vi "Dresden R2R Sputter 03.02.2018 IY24.vi"() -> ()   [LabVIEW 2009] (continued)
      }
    }
    n7249 = VISA Write(VISA resource name=w10738, write buffer=bytes[3], error in (no error)=w10737) -> (VISA resource name out=w10764, error out=w10763)  [unwired: 1 out]
    n7250 = stacked-sequence {
      tunnel: [w11051] -> w10740
      tunnel: w10764 -> [w11051]
      tunnel: [w11050] -> w10739
      tunnel: w10763 -> [w11050]
      frame #0 {
        n7251 = Wait Until Next ms Multiple(millisecond multiple=i32? 40) -> ()  [unwired: 1 out]
      }
    }
    n7252 = property class="Instr"(reference=w10740, error in=w10739) -> (reference out=w10766, error out=w10765, "Serial Settings:Number of Bytes at Serial Port"=w10767)
    n7253 = VISA Read(VISA resource name=w10766, byte count=w10767, error in (no error)=w10765) -> (VISA resource name out=w10736, read buffer=w10741, error out=w10735)  [unwired: 1 out]
    n7254 = Match Pattern(string=w10741, regular expression="Á") -> (after substring=w10731)  [unwired: 4 out]
    n7255 = String To Byte Array(string=w10731) -> (unsigned byte array=w10754)
    n7256 = String Length(string=w10731) -> (length=w10675)
    n7257 = Index Array(array=w10754, index=i32? 3) -> (element=w10746)
    n7258 = Index Array(array=w10754, index=i32? 2) -> (element=w10749)
    n7259 = Index Array(array=w10754, index=i32? 1) -> (element=w10758)
    n7260 = Index Array(array=w10754, index=data[5B]) -> (element=w10756)
    n7261 = Not Equal To 0?(x=w10675) -> (x != 0?=w10732)
    n7262 = To Unsigned Long Integer(number=w10746) -> (unsigned 32bit integer=w10748)
    n7263 = To Unsigned Long Integer(number=w10749) -> (unsigned 32bit integer=w10751)
    n7264 = To Unsigned Long Integer(number=w10758) -> (unsigned 32bit integer=w10757)
    n7265 = To Unsigned Long Integer(number=w10756) -> (unsigned 32bit integer=w10742)
    n7266 = case shown="True" w10732 {
      tunnel: [w11043 w11045] -> w10734
      tunnel: [w11042 w11044] -> w10733
      tunnel: w10736 -> [w11043 w11047]
      tunnel: w10735 -> [w11042 w11046]
      frame #0 {
      }
      frame #1 {
        n7267 = VISA Write(VISA resource name=w11047, write buffer=bytes[1], error in (no error)=w11046) -> (VISA resource name out=w11045, error out=w11044)  [unwired: 1 out]
      }
    }
    n7268 = Multiply(x=i32? 256, y=w10748) -> (x*y=w10745)
    n7269 = Multiply(x=i32? 256, y=w10751) -> (x*y=w10744)
    n7270 = Multiply(x=i32? 256, y=w10757) -> (x*y=w10743)
    n7271 = Compound Arithmetic op=ADD(w10745, w10744, w10743, w10742) -> (w10721)
    n7272 = case shown="1" w10675 {
      tunnel: w10721 -> [_ w11023]
      frame #0 {
      }
      frame #1 {
        "Frequency" <- w11023
      }
    }
  }
  n7273 = stacked-sequence {
    frame #0 {
      # "TM3"
      n7274 = stacked-sequence {
        tunnel: [_ "Thickness_Monitor3"] -> w11454
        frame #0 {
          n7275 = Wait (ms)(milliseconds to wait=u32 500) -> ()  [unwired: 1 out]
        }
        frame #1 {
        }
      }
      n7276 = call-poly "VISA Configure Serial Port"("VISA resource name"=w11454, "baud rate (9600)"=u32 57600) -> ("VISA resource name out"=w11456:refnum<visa-resource-name>, "error out"=w11455:errorcluster)  [unwired: 12 in]
      n7277 = VISA Clear(VISA resource name=w11456, error in (no error)=w11455) -> (VISA resource name out=w11453:refnum<visa-resource-name>, error out=w11452:errorcluster)
      n7278 = while {
        stop <- FALSE stop-if-true
        n7279 = local read "Tm3_fail"() -> (w11464:bool)
        n7280 = Wait Until Next ms Multiple(millisecond multiple=u32 1000) -> ()  [unwired: 1 out]
        n7281 = case shown="False" w11464 {
          frame #0 {
            # "Rate"
            n7282 = local read "Snsr3_thick"() -> (w11507:dbl)
            n7283 = feedback #159() -> (w11508:dbl)  [unwired: 1 in]
            n7284 = Subtract(x=w11507, y=w11508) -> (x-y=w11488:dbl)
            n7285 = local read "Material_density 3"() -> (w11489:dbl)
            n7286 = local read "Z_factor3"() -> (w11490:dbl)
            n7287 = feedback #160() -> (w11504:dbl)  [unwired: 1 in]
            n7288 = feedback #161() -> (w11492:dbl)  [unwired: 1 in]
            n7289 = feedback #162() -> (w11493:dbl)  [unwired: 1 in]
            n7290 = Equal?(x=w11492, y=w11490) -> (x = y?=w11494:bool)
            n7291 = Equal?(x=w11493, y=w11489) -> (x = y?=w11495:bool)
            n7292 = feedback #163() -> (w11503:dbl)  [unwired: 1 in]
            n7293 = And(x=w11494, y=w11495) -> (x .and. y?=w11491:bool)
            n7294 = case shown="True" w11491 {
              tunnel: w11488 -> [_ w11523]
              tunnel: [0.0 w11523] -> w11487
              frame #0 {
                n7295 = Wait (ms)(milliseconds to wait=u32 2000) -> ()  [unwired: 1 out]
              }
              frame #1 {
              }
            }
            n7296 = feedback #164() -> (w11502:dbl)  [unwired: 1 in]
            n7297 = feedback #165() -> (w11501:dbl)  [unwired: 1 in]
            n7298 = feedback #166() -> (w11500:dbl)  [unwired: 1 in]
            n7299 = feedback #167() -> (w11499:dbl)  [unwired: 1 in]
            n7300 = feedback #168() -> (w11498:dbl)  [unwired: 1 in]
            n7301 = feedback #169() -> (w11497:dbl)  [unwired: 1 in]
            n7302 = feedback #170() -> (w11496:dbl)  [unwired: 1 in]
            n7303 = Compound Arithmetic op=ADD(w11487, w11504, w11503, w11502, w11501, w11500, w11499, w11498, w11497, w11496) -> (w11505:dbl)
            n7304 = Divide(x=w11505, y=10.0) -> (x/y=w11484:dbl)
            n7305 = Greater Or Equal?(x=w11484, y=0.0) -> (x >= y?=w11486:bool)
            n7306 = case shown="True" w11486 {
              tunnel: w11484 -> [w11513 _]
              frame #0 {
                # "kA"
                n7307 = Divide(x="Tooling_factor3", y=100.0) -> (x/y=w11514:dbl)
                n7308 = Multiply(x=w11514, y=w11513) -> (x*y=w11509:dbl)
                "Rate3-2" <- w11509
                "Rate3-1" <- w11509
                "Rate3-3" <- w11509
                "Rate3-4" <- w11509
                "Rate3-5" <- w11509
                n7309 = Divide(x=w11509, y=1000.0) -> (x/y=w11518:dbl)
                n7310 = local read "Thickness 3-1"() -> (w11519:dbl)
                n7311 = Add(x=w11519, y=w11518) -> (x+y=w11511:dbl)
                n7312 = Greater?(x=w11511, y=0.0) -> (0:w11516:bool)
                n7313 = case shown="True" w11516 {
                  tunnel: w11511 -> [_ w11520]
                  frame #0 {
                  }
                  frame #1 {
                    "Thickness 3-1" <- w11520
                    "Thickness 3-2" <- w11520
                    "Thickness 3-3" <- w11520
                  }
                }
              }
              frame #1 {
              }
            }
          }
          frame #1 {
            w11524 = 0.0 ("Rate1-1")
            n7314 = local write "Rate3-1"(w11524) -> ()
            n7315 = local write "Rate3-2"(w11524) -> ()
            n7316 = local write "Rate3-3"(w11524) -> ()
            n7317 = local write "Rate3-4"(w11524) -> ()
            n7318 = local write "Rate3-5"(w11524) -> ()
          }
        }
        n7319 = Compound Arithmetic op=OR("Tm3_auto_set_zero", "Set3_zero_parameter", "Set3_zero_parameter2") -> (w11460:bool)
        n7320 = case shown="True" w11460 {
          frame #0 {
          }
          frame #1 {
            w11479 = 0.0 ("Thickness 1-1")
            n7321 = local read "Start_coating"() -> (w11474:bool)
            n7322 = local read "Semi"() -> (w11475:bool)
            n7323 = local read "Loading"() -> (w11473:bool)
            n7324 = Compound Arithmetic op=OR(w11475, w11474, w11473) -> (w11476:bool)
            n7325 = case shown="False" w11476 {
              frame #0 {
                n7326 = stacked-sequence {
                  frame #0 {
                    n7327 = local write "Pps_code_entry"("" ("Pps_code_entry")) -> ()
                  }
                  frame #1 {
                    n7328 = Wait (ms)(milliseconds to wait=u32 500) -> ()  [unwired: 1 out]
                  }
                  frame #2 {
                    n7329 = local write "Ppsok"(TRUE ("Ppsok")) -> ()
                  }
                }
              }
              frame #1 {
              }
            }
            n7330 = local write "Set3_zero_parameter2"(FALSE ("Set1_zero_parameter 2")) -> ()
            n7331 = local write "Set3_zero_parameter"(FALSE ("Set1_zero_parameter")) -> ()
            n7332 = local write "Tm3_auto_set_zero"(FALSE ("Tm1_auto_set_zero")) -> ()
            n7333 = local write "Thickness 3-2"(w11479) -> ()
            n7334 = local write "Thickness 3-3"(w11479) -> ()
          }
        }
        n7335 = local read "Frequency_short3"() -> (w11459:u32)
        n7336 = Not Equal To 0?(x=w11459) -> (x != 0?=w11458:bool)
        n7337 = case shown="True" w11458 {
          frame #0 {
            n7338 = local write "Tm3_gui"(FALSE ("Tm1_fail")) -> ()
          }
          frame #1 {
            n7339 = local read "Thickness 3-1"() -> (w11470:dbl)
            n7340 = Greater?(x=w11470, y="Thickness_for_TM3_gui") -> (0:w11468:bool)
            n7341 = case shown="False" w11468 {
              frame #0 {
                n7342 = local write "Tm3_gui"(FALSE ("Tm1_fail")) -> ()
              }
              frame #1 {
                n7343 = local write "Tm3_gui"(TRUE ("Tm1_fail")) -> ()
              }
            }
          }
        }
      }
      n7344 = while {
        tunnel: w11453 -> [w11677]
        tunnel: w11452 -> [w11676]
        tunnel: [w11670] -> w11451
        tunnel: [w11669] -> w11450
        stop <- FALSE stop-if-true
        n7345 = Wait Until Next ms Multiple(millisecond multiple=u32 250) -> ()  [unwired: 1 out]
        n7346 = case shown="True" "Tm3_set_parameters" {
          frame #0 {
          }
          frame #1 {
            n7347 = stacked-sequence {
              frame #0 {
                n7348 = local write "Pps_code_entry"("" ("Pps_code_entry")) -> ()
              }
              frame #1 {
                n7349 = Wait (ms)(milliseconds to wait=u32 500) -> ()  [unwired: 1 out]
              }
              frame #2 {
                n7350 = local write "Ppsok"(TRUE ("Ppsok")) -> ()
              }
            }
          }
        }
        n7351 = VISA Write(VISA resource name=w11677, write buffer="ª\u0004È¡È\u0001S\u0001\u0000\u0000\u0000Š", error in (no error)=w11676) -> (VISA resource name out=w11679:refnum<visa-resource-name>, error out=w11680:errorcluster)  [unwired: 1 out]
        n7352 = property class="Instr"(reference=w11679, error in=w11680) -> (reference out=w11681:refnum<visa-resource-name>, error out=w11683:errorcluster, "Serial Settings:Number of Bytes at Serial Port"=w11682:u32)
        n7353 = stacked-sequence {
          tunnel: [w11810] -> w11684
          tunnel: w11681 -> [w11810]
          tunnel: [w11809] -> w11686
          tunnel: w11683 -> [w11809]
          tunnel: [w11808] -> w11685
          tunnel: w11682 -> [w11808]
          frame #0 {
            n7354 = Wait (ms)(milliseconds to wait=u32 100) -> ()  [unwired: 1 out]
          }
        }
        n7355 = VISA Read(VISA resource name=w11684, byte count=w11685, error in (no error)=w11686) -> (VISA resource name out=w11670:refnum<visa-resource-name>, read buffer=w11671:string, error out=w11669:errorcluster)  [unwired: 1 out]
        "Tm3_read" <- w11671
        n7356 = String Length(string=w11671) -> (length=w11673:i32)
        n7357 = Greater Or Equal?(x=w11673, y=17) -> (x >= y?=w11672:bool)
        n7358 = case shown="True" w11672 {
          tunnel: w11671 -> [w11690 w11709]
          frame #0 {
            n7359 = String Length(string=w11690) -> (length=w11694:i32)
            n7360 = feedback #171() -> (w11693:bool)  [unwired: 1 in]
            n7361 = Equal To 0?(x=w11694) -> (x = 0?=w11691:bool)
            n7362 = case shown="True" w11691 {
              tunnel: [TRUE FALSE] -> w11692
              tunnel: w11693 -> [_ w11707]
              tunnel: [FALSE w11704] -> w11689
              frame #0 {
              }
              frame #1 {
                n7363 = call "Elapsed Time176"("Reset"=w11707) -> ("Elapsed Time (s)"=w11705:dbl)  [unwired: 11 in, 7 out]
                n7364 = Greater?(x=w11705, y=5.0) -> (0:w11704:bool)
              }
            }
            n7365 = case shown="True" w11689 {
              frame #0 {
                n7366 = local write "Tm3_Conn_err"(FALSE ("TM 1_err")) -> ()
              }
              frame #1 {
                n7367 = local write "Crystal3 Life Time :"(0.0 ("Crystal Life Time :")) -> ()
                n7368 = local write "Oscillator_status 3"(u32 0 ("Oscillator_status")) -> ()
                n7369 = local write "Frequency_long 3"(u32 0 ("Frequency_long")) -> ()
                n7370 = local write "Crystal3 Status :"("") -> ()
                n7371 = local write "Tm3_gui"(FALSE ("Tm1_gui")) -> ()
                "Tm3_Conn_err" <- TRUE ("Tm_Conn_err")
              }
            }
            n7372 = local write "Tm3_fail"(w11689) -> ()
          }
          frame #1 {
            # "hex"
            # "hex"
            # "hex"
            # "hex"
            # "hex"
            n7373 = local write "Tm3_Conn_err"(FALSE ("TM 1_err")) -> ()
            n7374 = Match Pattern(string=w11709, regular expression="ª\t\u0001¡ÈÈS") -> (before substring=w11737:string, after substring=w11738:string)  [unwired: 3 out]
            n7375 = Concatenate Strings(w11738, w11737) -> (w11714:string)
            "Combined_read3" <- w11714
            n7376 = String Subset(string=w11714, offset (0)=4, length (rest)=1 ("length (rest)")) -> (substring=w11715:string)
            n7377 = String Subset(string=w11714, offset (0)=5 ("offset (0) 2"), length (rest)=1 ("length (rest)")) -> (substring=w11716:string)
            n7378 = String Subset(string=w11714, offset (0)=0 ("offset (0) 5"), length (rest)=4 ("length (rest)")) -> (substring=w11731:string)
            n7379 = String Subset(string=w11714, offset (0)=6 ("offset (0) 3"), length (rest)=2 ("length (rest)")) -> (substring=w11717:string)
            n7380 = String Subset(string=w11714, offset (0)=8 ("offset (0) 4"), length (rest)=1 ("length (rest)")) -> (substring=w11718:string)
            n7381 = String To Byte Array(string=w11715) -> (unsigned byte array=w11729:u8[])
            n7382 = String To Byte Array(string=w11717) -> (unsigned byte array=w11723:u8[])
            n7383 = String To Byte Array(string=w11731) -> (unsigned byte array=w11712:u8[])
            n7384 = String To Byte Array(string=w11718) -> (unsigned byte array=w11721:u8[])
            n7385 = String To Byte Array(string=w11716) -> (unsigned byte array=w11727:u8[])
            n7386 = for {
              shift-right: [w11800] -> w11728
              shift-left: "" -> [w11798]
              tunnel: w11729 -> [w11804] mode=indexing
              n7387 = Number To Hexadecimal String(2:w11804) -> (0:w11801:string)  [unwired: 1 in]
              n7388 = String Length(string=w11801) -> (length=w11803:i32)
              n7389 = Less?(x=w11803, y=2) -> (x < y?=w11794:bool)
              n7390 = Select(t="0" ("format string"), s=w11794, f="") -> (s? t:f=w11796:string)
              n7391 = Concatenate Strings(w11796, w11801) -> (w11799:string)
              n7392 = Concatenate Strings(w11798, w11799) -> (w11800:string)
            }
            n7393 = for {
              shift-right: [w11778] -> w11722
              shift-left: "" -> [w11776]
              tunnel: w11723 -> [w11782] mode=indexing
              n7394 = Number To Hexadecimal String(2:w11782) -> (0:w11779:string)  [unwired: 1 in]
              n7395 = String Length(string=w11779) -> (length=w11781:i32)
              n7396 = Less?(x=w11781, y=2) -> (x < y?=w11772:bool)
              n7397 = Select(t="0" ("format string"), s=w11772, f="") -> (s? t:f=w11774:string)
              n7398 = Concatenate Strings(w11774, w11779) -> (w11777:string)
              n7399 = Concatenate Strings(w11776, w11777) -> (w11778:string)
            }
            n7400 = for {
              shift-right: [w11756] -> w11711
              shift-left: "" -> [w11754]
              tunnel: w11712 -> [w11760] mode=indexing
              n7401 = Number To Hexadecimal String(2:w11760) -> (0:w11757:string)  [unwired: 1 in]
              n7402 = String Length(string=w11757) -> (length=w11759:i32)
              n7403 = Less?(x=w11759, y=2) -> (x < y?=w11750:bool)
              n7404 = Select(t="0" ("format string"), s=w11750, f="") -> (s? t:f=w11752:string)
              n7405 = Concatenate Strings(w11752, w11757) -> (w11755:string)
              n7406 = Concatenate Strings(w11754, w11755) -> (w11756:string)
            }
            n7407 = for {
              shift-right: [w11767] -> w11719
              shift-left: "" -> [w11765]
              tunnel: w11721 -> [w11771] mode=indexing
              n7408 = Number To Hexadecimal String(2:w11771) -> (0:w11768:string)  [unwired: 1 in]
              n7409 = String Length(string=w11768) -> (length=w11770:i32)
              n7410 = Less?(x=w11770, y=2) -> (x < y?=w11761:bool)
              n7411 = Select(t="0" ("format string"), s=w11761, f="") -> (s? t:f=w11763:string)
              n7412 = Concatenate Strings(w11763, w11768) -> (w11766:string)
              n7413 = Concatenate Strings(w11765, w11766) -> (w11767:string)
            }
            n7414 = for {
              shift-right: [w11789] -> w11725
              shift-left: "" -> [w11787]
              tunnel: w11727 -> [w11793] mode=indexing
              n7415 = Number To Hexadecimal String(2:w11793) -> (0:w11790:string)  [unwired: 1 in]
              n7416 = String Length(string=w11790) -> (length=w11792:i32)
              n7417 = Less?(x=w11792, y=2) -> (x < y?=w11783:bool)
              n7418 = Select(t="0" ("format string"), s=w11783, f="") -> (s? t:f=w11785:string)
              n7419 = Concatenate Strings(w11785, w11790) -> (w11788:string)
              n7420 = Concatenate Strings(w11787, w11788) -> (w11789:string)
            }
            n7421 = Hexadecimal String To Number(string=w11722) -> (number=→"Measurement_time 3":u32)  [unwired: 2 in, 1 out]
            n7422 = Hexadecimal String To Number(string=w11725) -> (number=→"Sample_number 3":u32)  [unwired: 2 in, 1 out]
            n7423 = Hexadecimal String To Number(string=w11728) -> (number=→"Oscillator_status 3":u32)  [unwired: 2 in, 1 out]
            n7424 = Hexadecimal String To Number(string=w11711) -> (number=→"Frequency_long 3":u32)  [unwired: 2 in, 1 out]
            n7425 = Hexadecimal String To Number(string=w11719) -> (number=→"Device_ID 3":u32)  [unwired: 2 in, 1 out]
          }
        }
      }
      n7426 = VISA Close(VISA resource name=w11451, error in (no error)=w11450) -> ()  [unwired: 1 out]
      n7427 = while {
        stop <- FALSE stop-if-true
        w11546 = 6000000.0 ("Fq")
        w11529 = 3.141592653589793
        # "cm"
        # "Tickness \n    (cm)"
        # "density of quartz \n2.648 g/cm3"
        # "Frequency constants \n1.668 E+5 Hz · cm"
        # "Frequency Of Loaded \nSensor Crystal"
        # "Si02 Acoustic Impedance"
        # "Si02 Acoustic Impedance"
        n7428 = local read "Frequency_short3"() -> (w11526:u32)
        n7429 = Wait Until Next ms Multiple(millisecond multiple=u32 250) -> ()  [unwired: 1 out]
        n7430 = local read "Tm3_read"() -> (w11554:string)
        n7431 = local read "Oscillator_status 3"() -> (w11548:u32)
        n7432 = local read "Frequency_long 3"() -> (w11551:u32)
        n7433 = Equal?(x=w11554, y="") -> (x = y?=w11553:bool)
        n7434 = case shown="False" w11553 {
          tunnel: w11526 -> [_ _]
          tunnel: w11548 -> [w11593 _]
          tunnel: w11526 -> [w11592 _]
          frame #0 {
            n7435 = Equal To 0?(x=w11593) -> (x = 0?=w11618:bool)
            n7436 = feedback #172() -> (w11615:bool)  [unwired: 1 in]
            n7437 = feedback #173() -> (w11613:bool)  [unwired: 1 in]
            n7438 = Less Or Equal?(x=w11592, y=4500000 ("lower limit")) -> (x <= y?=w11617:bool)
            n7439 = case shown="True" w11618 {
              tunnel: [TRUE FALSE] -> w11616
              tunnel: w11615 -> [_ w11660]
              tunnel: [FALSE w11657] -> w11600
              frame #0 {
              }
              frame #1 {
                n7440 = call "Elapsed Time178"("Reset"=w11660) -> ("Elapsed Time (s)"=w11658:dbl)  [unwired: 11 in, 7 out]
                n7441 = Greater?(x=w11658, y=5.0) -> (0:w11657:bool)
              }
            }
            n7442 = case shown="True" w11617 {
              tunnel: [TRUE FALSE] -> w11614
              tunnel: w11613 -> [_ w11667]
              tunnel: [FALSE w11664] -> w11599
              frame #0 {
              }
              frame #1 {
                n7443 = call "Elapsed Time177"("Reset"=w11667) -> ("Elapsed Time (s)"=w11665:dbl)  [unwired: 11 in, 7 out]
                n7444 = Greater?(x=w11665, y=5.0) -> (0:w11664:bool)
              }
            }
            n7445 = Or(x=w11600, y=w11599) -> (x .or. y?=w11595:bool)
            n7446 = Subtract(x=100.0, y="Warning 3 limit") -> (x-y=w11612:dbl)
            n7447 = Multiply(x=w11612, y=1500000.0) -> (x*y=w11610:dbl)
            n7448 = Divide(x=w11610, y=100.0) -> (x/y=w11607:dbl)
            n7449 = Subtract(x=6000000.0, y=w11607) -> (x-y=w11602:dbl)
            n7450 = feedback #174() -> (w11603:bool)  [unwired: 1 in]
            n7451 = Less Or Equal?(x=w11592, y=w11602) -> (x <= y?=w11604:bool)
            n7452 = case shown="True" w11604 {
              tunnel: [TRUE FALSE] -> w11601
              tunnel: w11603 -> [_ w11653]
              tunnel: [FALSE w11650] -> w11596
              frame #0 {
              }
              frame #1 {
                n7453 = call "Elapsed Time179"("Reset"=w11653) -> ("Elapsed Time (s)"=w11651:dbl)  [unwired: 11 in, 7 out]
                n7454 = Greater?(x=w11651, y=5.0) -> (0:w11650:bool)
              }
            }
            n7455 = case shown="False" w11596 {
              tunnel: [w11624 "Fail" ("Crystal Status :")] -> w11598
              tunnel: [w11623 0.0 ("Crystal Life Time : 2")] -> w11597
              tunnel: w11592 -> [w11622 _]
              tunnel: w11595 -> [w11621 _]
              tunnel: [w11620 TRUE ("Tm1_fail")] -> w11594
              frame #0 {
                n7456 = case shown="False" w11621 {
                  tunnel: ["Good" ("Crystal Status :") "Fail" ("Crystal Status :")] -> w11624
                  tunnel: [w11628 0.0 ("Crystal Life Time : 2")] -> w11623
                  tunnel: w11622 -> [w11627 _]
                  tunnel: [FALSE ("Tm1_fail") TRUE ("Tm1_fail")] -> w11620
                  frame #0 {
                    n7457 = local write "Tm3_Crys_err"(FALSE ("Tm1_Crys_err")) -> ()
                    n7458 = In Range and Coerce(upper limit=6000000, x=w11627, lower limit=4500000) -> (coerced(x)=w11637:u32)  [unwired: 1 out]
                    n7459 = Subtract(x=6000000.0, y=w11637) -> (x-y=w11630:dbl)
                    n7460 = Multiply(x=w11630, y=100.0) -> (x*y=w11632:dbl)
                    n7461 = Divide(x=w11632, y=1500000.0) -> (x/y=w11633:dbl)
                    n7462 = Subtract(x=100.0, y=w11633) -> (x-y=w11628:dbl)
                    "Crystal3_Real" <- w11628
                  }
                  frame #1 {
                    "Tm3_Crys_err" <- TRUE ("Tm1_Cry_err")
                  }
                }
              }
              frame #1 {
                n7463 = local write "Tm3_Crys_err"(TRUE ("Tm1_Crys_err")) -> ()
              }
            }
            "Crystal3 Status :" <- w11598
            "Crystal3 Life Time :" <- w11597
            "Crystal3 Life Time : 2" <- w11597
            n7464 = local write "Tm3_fail"(w11594) -> ()
          }
          frame #1 {
          }
        }
        n7465 = Equal To 0?(x=w11551) -> (x = 0?=w11552:bool)
        n7466 = case shown="False" w11552 {
          tunnel: w11551 -> [w11565 _]
          frame #0 {
            n7467 = Number To Decimal String(number=w11565) -> (decimal integer string=w11567:string)  [unwired: 1 in]
            n7468 = String Subset(string=w11567, offset (0)=0, length (rest)=7 ("length (rest)")) -> (substring=w11566:string)
            n7469 = Decimal String To Number(string=w11566) -> (number=w11559:i32)  [unwired: 2 in, 1 out]
            n7470 = Less?(x=w11559, y=4500000 ("lower limit")) -> (x < y?=w11563:bool)
            n7471 = feedback #175() -> (w11561:bool)  [unwired: 1 in]
            n7472 = case shown="True" w11563 {
              tunnel: [TRUE FALSE] -> w11562
              tunnel: w11561 -> [_ w11589]
              tunnel: [FALSE w11586] -> w11560
              frame #0 {
              }
              frame #1 {
                n7473 = call "Elapsed Time180"("Reset"=w11589) -> ("Elapsed Time (s)"=w11587:dbl)  [unwired: 11 in, 7 out]
                n7474 = Greater?(x=w11587, y=20.0) -> (0:w11586:bool)
              }
            }
            n7475 = case shown="False" w11560 {
              tunnel: w11559 -> [w11570 _]
              frame #0 {
                n7476 = Greater?(x=w11570, y=4500000 ("lower limit")) -> (0:w11573:bool)
                n7477 = Less Or Equal?(x=w11570, y=6000000 ("lower limit")) -> (x <= y?=w11571:bool)
                n7478 = And(x=w11573, y=w11571) -> (x .and. y?=w11572:bool)
                n7479 = case shown="True" w11572 {
                  tunnel: w11570 -> [_ w11576]
                  frame #0 {
                  }
                  frame #1 {
                    n7480 = feedback #176() -> (w11578:i32)  [unwired: 1 in]
                    n7481 = Subtract(x=w11578, y=w11576) -> (x-y=w11580:i32)
                    n7482 = Less?(x=w11580, y=200) -> (x < y?=w11577:bool)
                    n7483 = case shown="True" w11577 {
                      tunnel: w11576 -> [_ w11581]
                      tunnel: w11576 -> [_ _]
                      frame #0 {
                      }
                      frame #1 {
                        "Frequency_short3" <- w11581
                      }
                    }
                  }
                }
              }
              frame #1 {
                n7484 = local write "Tm3_fail"(TRUE ("Tm1_fail")) -> ()
                n7485 = local write "Frequency_short3"(u32 0 ("Frequency_short")) -> ()
              }
            }
          }
          frame #1 {
            n7486 = local write "Frequency_short3"(u32 0 ("Frequency_short")) -> ()
          }
        }
        n7487 = Divide(x=8.83, y="Z_factor3") -> (x/y=w11530:dbl)
        n7488 = Subtract(x=w11546, y=w11526) -> (x-y=w11547:dbl)
        n7489 = Divide(x=w11547, y=w11546) -> (x/y=w11545:dbl)
        n7490 = Multiply(x=w11545, y=w11529) -> (x*y=w11544:dbl)
        n7491 = Tangent(1:w11544) -> (0:w11543:dbl)
        n7492 = Multiply(x=w11543, y=w11530) -> (x*y=w11533:dbl)
        n7493 = Inverse Tangent(1:w11533) -> (0:w11532:dbl)
        n7494 = Multiply(x=w11532, y=2.648 ("Pq")) -> (x*y=w11541:dbl)
        n7495 = Multiply(x=w11541, y=166800.0 ("Nq")) -> (x*y=w11539:dbl)
        n7496 = Divide(x=w11539, y=w11529) -> (x/y=w11538:dbl)
        n7497 = Divide(x=w11538, y="Material_density 3") -> (x/y=w11537:dbl)
        n7498 = Divide(x=w11537, y=w11530) -> (x/y=w11536:dbl)
        n7499 = Divide(x=w11536, y=w11526) -> (x/y=w11534:dbl)
        n7500 = Multiply(x=w11534, y=100000000.0) -> (x*y=w11525:dbl)
        n7501 = Greater?(x=w11525, y=0.0) -> (0:w11527:bool)
        n7502 = case shown="True" w11527 {
          tunnel: w11525 -> [_ w11558]
          frame #0 {
          }
          frame #1 {
            "Snsr3_thick" <- w11558
          }
        }
      }
    }
  }
  n7503 = call <vilib>:"MB Serial Init.vi"("Timeout"=i32? 2000, "Mode"=w767, "Parity"=w769, "Baud Rate"=i32? 9600, "VISA resource name"="Moxa I/O Ch 2") -> ("error out"=w772:errorcluster, "VISA resource name out"=w746:refnum<visa-resource-name>)  [unwired: 2 in, 3 out]
  n7504 = stacked-sequence {
    frame #0 {
      # "TM1"
      n7505 = stacked-sequence {
        tunnel: [_ "Thickness_Monitor1"] -> w11818
        frame #0 {
          n7506 = Wait (ms)(milliseconds to wait=u32 500) -> ()  [unwired: 1 out]
        }
        frame #1 {
        }
      }
      n7507 = call-poly "VISA Configure Serial Port"("VISA resource name"=w11818, "baud rate (9600)"=u32 57600) -> ("VISA resource name out"=w11820:refnum<visa-resource-name>, "error out"=w11819:errorcluster)  [unwired: 12 in]
      n7508 = VISA Clear(VISA resource name=w11820, error in (no error)=w11819) -> (VISA resource name out=w11817:refnum<visa-resource-name>, error out=w11816:errorcluster)
      n7509 = while {
        stop <- FALSE stop-if-true
        n7510 = local read "Tm1_fail"() -> (w11828:bool)
        n7511 = Wait Until Next ms Multiple(millisecond multiple=u32 1000) -> ()  [unwired: 1 out]
        n7512 = case shown="False" w11828 {
          frame #0 {
            # "Rate"
            n7513 = local read "Snsr_thick"() -> (w11871:dbl)
            n7514 = feedback #177() -> (w11872:dbl)  [unwired: 1 in]
            n7515 = Subtract(x=w11871, y=w11872) -> (x-y=w11852:dbl)
            n7516 = local read "Material_density"() -> (w11853:dbl)
            n7517 = local read "Z_factor"() -> (w11854:dbl)
            n7518 = feedback #178() -> (w11868:dbl)  [unwired: 1 in]
            n7519 = feedback #179() -> (w11856:dbl)  [unwired: 1 in]
            n7520 = feedback #180() -> (w11857:dbl)  [unwired: 1 in]
            n7521 = Equal?(x=w11856, y=w11854) -> (x = y?=w11858:bool)
            n7522 = Equal?(x=w11857, y=w11853) -> (x = y?=w11859:bool)
            n7523 = feedback #181() -> (w11867:dbl)  [unwired: 1 in]
            n7524 = And(x=w11858, y=w11859) -> (x .and. y?=w11855:bool)
            n7525 = case shown="True" w11855 {
              tunnel: w11852 -> [_ w11887]
              tunnel: [0.0 w11887] -> w11851
              frame #0 {
                n7526 = Wait (ms)(milliseconds to wait=u32 2000) -> ()  [unwired: 1 out]
              }
              frame #1 {
              }
            }
            n7527 = feedback #182() -> (w11866:dbl)  [unwired: 1 in]
            n7528 = feedback #183() -> (w11865:dbl)  [unwired: 1 in]
            n7529 = feedback #184() -> (w11864:dbl)  [unwired: 1 in]
            n7530 = feedback #185() -> (w11863:dbl)  [unwired: 1 in]
            n7531 = feedback #186() -> (w11862:dbl)  [unwired: 1 in]
            n7532 = feedback #187() -> (w11861:dbl)  [unwired: 1 in]
            n7533 = feedback #188() -> (w11860:dbl)  [unwired: 1 in]
            n7534 = Compound Arithmetic op=ADD(w11851, w11868, w11867, w11866, w11865, w11864, w11863, w11862, w11861, w11860) -> (w11869:dbl)
            n7535 = Divide(x=w11869, y=10.0) -> (x/y=w11848:dbl)
            n7536 = Greater Or Equal?(x=w11848, y=0.0) -> (x >= y?=w11850:bool)
            n7537 = case shown="True" w11850 {
              tunnel: w11848 -> [w11877 _]
              frame #0 {
                # "kA"
                n7538 = Divide(x="Tooling_factor1", y=100.0) -> (x/y=w11878:dbl)
                n7539 = Multiply(x=w11878, y=w11877) -> (x*y=w11873:dbl)
                "Rate1-2" <- w11873
                "Rate1-1" <- w11873
                "Rate 1-3" <- w11873
                "Rate 1-4" <- w11873
                "Rate 1-5" <- w11873
                n7540 = Divide(x=w11873, y=1000.0) -> (x/y=w11882:dbl)
                n7541 = local read "Thickness 1-1"() -> (w11883:dbl)
                n7542 = Add(x=w11883, y=w11882) -> (x+y=w11875:dbl)
                n7543 = Greater?(x=w11875, y=0.0) -> (0:w11880:bool)
                n7544 = case shown="True" w11880 {
                  tunnel: w11875 -> [_ w11884]
                  frame #0 {
                  }
                  frame #1 {
                    "Thickness 1-1" <- w11884
                    "Thickness 1-2" <- w11884
                    "Thickness 1-3" <- w11884
                  }
                }
              }
              frame #1 {
              }
            }
          }
          frame #1 {
            w11888 = 0.0 ("Rate1-1")
            n7545 = local write "Rate1-1"(w11888) -> ()
            n7546 = local write "Rate1-2"(w11888) -> ()
            n7547 = local write "Rate 1-3"(w11888) -> ()
            n7548 = local write "Rate 1-4"(w11888) -> ()
            n7549 = local write "Rate 1-5"(w11888) -> ()
          }
        }
        n7550 = Compound Arithmetic op=OR("Tm1_auto_set_zero", "Set1_zero_parameter", "Set1_zero_parameter 2") -> (w11824:bool)
        n7551 = case shown="True" w11824 {
          frame #0 {
          }
          frame #1 {
            w11843 = 0.0 ("Thickness 1-1")
            n7552 = local read "Start_coating"() -> (w11838:bool)
            n7553 = local read "Semi"() -> (w11839:bool)
            n7554 = local read "Loading"() -> (w11837:bool)
            n7555 = Compound Arithmetic op=OR(w11839, w11838, w11837) -> (w11840:bool)
            n7556 = case shown="False" w11840 {
              frame #0 {
                n7557 = stacked-sequence {
                  frame #0 {
                    n7558 = local write "Pps_code_entry"("" ("Pps_code_entry")) -> ()
                  }
                  frame #1 {
                    n7559 = Wait (ms)(milliseconds to wait=u32 500) -> ()  [unwired: 1 out]
                  }
                  frame #2 {
                    n7560 = local write "Ppsok"(TRUE ("Ppsok")) -> ()
                  }
                }
              }
              frame #1 {
              }
            }
            n7561 = local write "Set1_zero_parameter 2"(FALSE ("Set1_zero_parameter 2")) -> ()
            n7562 = local write "Set1_zero_parameter"(FALSE ("Set1_zero_parameter")) -> ()
            n7563 = local write "Tm1_auto_set_zero"(FALSE ("Tm1_auto_set_zero")) -> ()
            n7564 = local write "Thickness 1-2"(w11843) -> ()
            n7565 = local write "Thickness 1-3"(w11843) -> ()
          }
        }
        n7566 = local read "Frequency_short"() -> (w11823:u32)
        n7567 = Not Equal To 0?(x=w11823) -> (x != 0?=w11822:bool)
        n7568 = case shown="True" w11822 {
          frame #0 {
            n7569 = local write "Tm1_gui"(FALSE ("Tm1_fail")) -> ()
          }
          frame #1 {
            n7570 = local read "Thickness 1-1"() -> (w11834:dbl)
            n7571 = Greater?(x=w11834, y="Thickness_for_TM1_gui") -> (0:w11832:bool)
            n7572 = case shown="True" w11832 {
              frame #0 {
                n7573 = local write "Tm1_gui"(FALSE ("Tm1_fail")) -> ()
              }
              frame #1 {
                n7574 = local write "Tm1_gui"(TRUE ("Tm1_fail")) -> ()
              }
            }
          }
        }
      }
      n7575 = while {
        tunnel: w11817 -> [w12041]
        tunnel: w11816 -> [w12040]
        tunnel: [w12034] -> w11815
        tunnel: [w12033] -> w11814
        stop <- FALSE stop-if-true
        n7576 = Wait Until Next ms Multiple(millisecond multiple=u32 250) -> ()  [unwired: 1 out]
        n7577 = case shown="True" "Tm_set_parameters" {
          frame #0 {
          }
          frame #1 {
            n7578 = stacked-sequence {
              frame #0 {
                n7579 = local write "Pps_code_entry"("" ("Pps_code_entry")) -> ()
              }
              frame #1 {
                n7580 = Wait (ms)(milliseconds to wait=u32 500) -> ()  [unwired: 1 out]
              }
              frame #2 {
                n7581 = local write "Ppsok"(TRUE ("Ppsok")) -> ()
              }
            }
          }
        }
        n7582 = VISA Write(VISA resource name=w12041, write buffer="ª\u0004È¡È\u0001S\u0001\u0000\u0000\u0000Š", error in (no error)=w12040) -> (VISA resource name out=w12043:refnum<visa-resource-name>, error out=w12044:errorcluster)  [unwired: 1 out]
        n7583 = property class="Instr"(reference=w12043, error in=w12044) -> (reference out=w12045:refnum<visa-resource-name>, error out=w12047:errorcluster, "Serial Settings:Number of Bytes at Serial Port"=w12046:u32)
        n7584 = stacked-sequence {
          tunnel: [w12174] -> w12048
          tunnel: w12045 -> [w12174]
          tunnel: [w12173] -> w12050
          tunnel: w12047 -> [w12173]
          tunnel: [w12172] -> w12049
          tunnel: w12046 -> [w12172]
          frame #0 {
            n7585 = Wait (ms)(milliseconds to wait=u32 100) -> ()  [unwired: 1 out]
          }
        }
        n7586 = VISA Read(VISA resource name=w12048, byte count=w12049, error in (no error)=w12050) -> (VISA resource name out=w12034:refnum<visa-resource-name>, read buffer=w12035:string, error out=w12033:errorcluster)  [unwired: 1 out]
        "Tm_read" <- w12035
        n7587 = String Length(string=w12035) -> (length=w12037:i32)
        n7588 = Greater Or Equal?(x=w12037, y=17) -> (x >= y?=w12036:bool)
        n7589 = case shown="False" w12036 {
          tunnel: w12035 -> [w12054 w12073]
          frame #0 {
            n7590 = String Length(string=w12054) -> (length=w12058:i32)
            n7591 = feedback #189() -> (w12057:bool)  [unwired: 1 in]
            n7592 = Equal To 0?(x=w12058) -> (x = 0?=w12055:bool)
            n7593 = case shown="True" w12055 {
              tunnel: [TRUE FALSE] -> w12056
              tunnel: w12057 -> [_ w12071]
              tunnel: [FALSE w12068] -> w12053
              frame #0 {
              }
              frame #1 {
                n7594 = call "Elapsed Time166"("Reset"=w12071) -> ("Elapsed Time (s)"=w12069:dbl)  [unwired: 11 in, 7 out]
                n7595 = Greater?(x=w12069, y=5.0) -> (0:w12068:bool)
              }
            }
            n7596 = case shown="False" w12053 {
              frame #0 {
                n7597 = local write "Tm_Conn_err"(FALSE ("TM 1_err")) -> ()
              }
              frame #1 {
                n7598 = local write "Crystal Life Time :"(0.0 ("Crystal Life Time :")) -> ()
                n7599 = local write "Oscillator_status"(u32 0 ("Oscillator_status")) -> ()
                n7600 = local write "Frequency_long"(u32 0 ("Frequency_long")) -> ()
                n7601 = local write "Crystal Status :"("") -> ()
                n7602 = local write "Tm1_gui"(FALSE ("Tm1_gui")) -> ()
                "Tm_Conn_err" <- TRUE ("Tm_Conn_err")
              }
            }
            n7603 = local write "Tm1_fail"(w12053) -> ()
          }
          frame #1 {
            # "hex"
            # "hex"
            # "hex"
            # "hex"
            # "hex"
            n7604 = local write "Tm_Conn_err"(FALSE ("TM 1_err")) -> ()
            n7605 = Match Pattern(string=w12073, regular expression="ª\t\u0001¡ÈÈS") -> (before substring=w12101:string, after substring=w12102:string)  [unwired: 3 out]
            n7606 = Concatenate Strings(w12102, w12101) -> (w12078:string)
            "Combined_read" <- w12078
            n7607 = String Subset(string=w12078, offset (0)=4, length (rest)=1 ("length (rest)")) -> (substring=w12079:string)
            n7608 = String Subset(string=w12078, offset (0)=5 ("offset (0) 2"), length (rest)=1 ("length (rest)")) -> (substring=w12080:string)
            n7609 = String Subset(string=w12078, offset (0)=0 ("offset (0) 5"), length (rest)=4 ("length (rest)")) -> (substring=w12095:string)
            n7610 = String Subset(string=w12078, offset (0)=6 ("offset (0) 3"), length (rest)=2 ("length (rest)")) -> (substring=w12081:string)
            n7611 = String Subset(string=w12078, offset (0)=8 ("offset (0) 4"), length (rest)=1 ("length (rest)")) -> (substring=w12082:string)
            n7612 = String To Byte Array(string=w12079) -> (unsigned byte array=w12093:u8[])
            n7613 = String To Byte Array(string=w12081) -> (unsigned byte array=w12087:u8[])
            n7614 = String To Byte Array(string=w12095) -> (unsigned byte array=w12076:u8[])
            n7615 = String To Byte Array(string=w12082) -> (unsigned byte array=w12085:u8[])
            n7616 = String To Byte Array(string=w12080) -> (unsigned byte array=w12091:u8[])
            n7617 = for {
              shift-right: [w12164] -> w12092
              shift-left: "" -> [w12162]
              tunnel: w12093 -> [w12168] mode=indexing
              n7618 = Number To Hexadecimal String(2:w12168) -> (0:w12165:string)  [unwired: 1 in]
              n7619 = String Length(string=w12165) -> (length=w12167:i32)
              n7620 = Less?(x=w12167, y=2) -> (x < y?=w12158:bool)
              n7621 = Select(t="0" ("format string"), s=w12158, f="") -> (s? t:f=w12160:string)
              n7622 = Concatenate Strings(w12160, w12165) -> (w12163:string)
              n7623 = Concatenate Strings(w12162, w12163) -> (w12164:string)
            }
            n7624 = for {
              shift-right: [w12142] -> w12086
              shift-left: "" -> [w12140]
              tunnel: w12087 -> [w12146] mode=indexing
              n7625 = Number To Hexadecimal String(2:w12146) -> (0:w12143:string)  [unwired: 1 in]
              n7626 = String Length(string=w12143) -> (length=w12145:i32)
              n7627 = Less?(x=w12145, y=2) -> (x < y?=w12136:bool)
              n7628 = Select(t="0" ("format string"), s=w12136, f="") -> (s? t:f=w12138:string)
              n7629 = Concatenate Strings(w12138, w12143) -> (w12141:string)
              n7630 = Concatenate Strings(w12140, w12141) -> (w12142:string)
            }
            n7631 = for {
              shift-right: [w12120] -> w12075
              shift-left: "" -> [w12118]
              tunnel: w12076 -> [w12124] mode=indexing
              n7632 = Number To Hexadecimal String(2:w12124) -> (0:w12121:string)  [unwired: 1 in]
              n7633 = String Length(string=w12121) -> (length=w12123:i32)
              n7634 = Less?(x=w12123, y=2) -> (x < y?=w12114:bool)
              n7635 = Select(t="0" ("format string"), s=w12114, f="") -> (s? t:f=w12116:string)
              n7636 = Concatenate Strings(w12116, w12121) -> (w12119:string)
              n7637 = Concatenate Strings(w12118, w12119) -> (w12120:string)
            }
            n7638 = for {
              shift-right: [w12131] -> w12083
              shift-left: "" -> [w12129]
              tunnel: w12085 -> [w12135] mode=indexing
              n7639 = Number To Hexadecimal String(2:w12135) -> (0:w12132:string)  [unwired: 1 in]
              n7640 = String Length(string=w12132) -> (length=w12134:i32)
              n7641 = Less?(x=w12134, y=2) -> (x < y?=w12125:bool)
              n7642 = Select(t="0" ("format string"), s=w12125, f="") -> (s? t:f=w12127:string)
              n7643 = Concatenate Strings(w12127, w12132) -> (w12130:string)
              n7644 = Concatenate Strings(w12129, w12130) -> (w12131:string)
            }
            n7645 = for {
              shift-right: [w12153] -> w12089
              shift-left: "" -> [w12151]
              tunnel: w12091 -> [w12157] mode=indexing
              n7646 = Number To Hexadecimal String(2:w12157) -> (0:w12154:string)  [unwired: 1 in]
              n7647 = String Length(string=w12154) -> (length=w12156:i32)
              n7648 = Less?(x=w12156, y=2) -> (x < y?=w12147:bool)
              n7649 = Select(t="0" ("format string"), s=w12147, f="") -> (s? t:f=w12149:string)
              n7650 = Concatenate Strings(w12149, w12154) -> (w12152:string)
              n7651 = Concatenate Strings(w12151, w12152) -> (w12153:string)
            }
            n7652 = Hexadecimal String To Number(string=w12086) -> (number=→"Measurement_time":u32)  [unwired: 2 in, 1 out]
            n7653 = Hexadecimal String To Number(string=w12089) -> (number=→"Sample_number":u32)  [unwired: 2 in, 1 out]
            n7654 = Hexadecimal String To Number(string=w12092) -> (number=→"Oscillator_status":u32)  [unwired: 2 in, 1 out]
            n7655 = Hexadecimal String To Number(string=w12075) -> (number=→"Frequency_long":u32)  [unwired: 2 in, 1 out]
            n7656 = Hexadecimal String To Number(string=w12083) -> (number=→"Device_ID":u32)  [unwired: 2 in, 1 out]
          }
        }
      }
      n7657 = VISA Close(VISA resource name=w11815, error in (no error)=w11814) -> ()  [unwired: 1 out]
      n7658 = while {
        stop <- FALSE stop-if-true
        w11910 = 6000000.0 ("Fq")
        w11893 = 3.141592653589793
        # "cm"
        # "Tickness \n    (cm)"
        # "density of quartz \n2.648 g/cm3"
        # "Frequency constants \n1.668 E+5 Hz · cm"
        # "Frequency Of Loaded \nSensor Crystal"
        # "Si02 Acoustic Impedance"
        # "Si02 Acoustic Impedance"
        n7659 = local read "Frequency_short"() -> (w11890:u32)
        n7660 = Wait Until Next ms Multiple(millisecond multiple=u32 250) -> ()  [unwired: 1 out]
        n7661 = local read "Tm_read"() -> (w11918:string)
        n7662 = local read "Oscillator_status"() -> (w11912:u32)
        n7663 = local read "Frequency_long"() -> (w11915:u32)
        n7664 = Equal?(x=w11918, y="") -> (x = y?=w11917:bool)
        n7665 = case shown="False" w11917 {
          tunnel: w11890 -> [_ _]
          tunnel: w11912 -> [w11957 _]
          tunnel: w11890 -> [w11956 _]